vi "9_3.vi"() -> ()   [LabVIEW 2026]
panel:
  out "spreadsheet string":string
  in  "format string":string
  out "text 3":string
  in  "file path (use dialog) 4":path
  in  "file path (use dialog) 3":path
  in  "file path (use dialog) 2":path
  in  "text 2":string
  out "text":string
  in  "file path (use dialog)":path
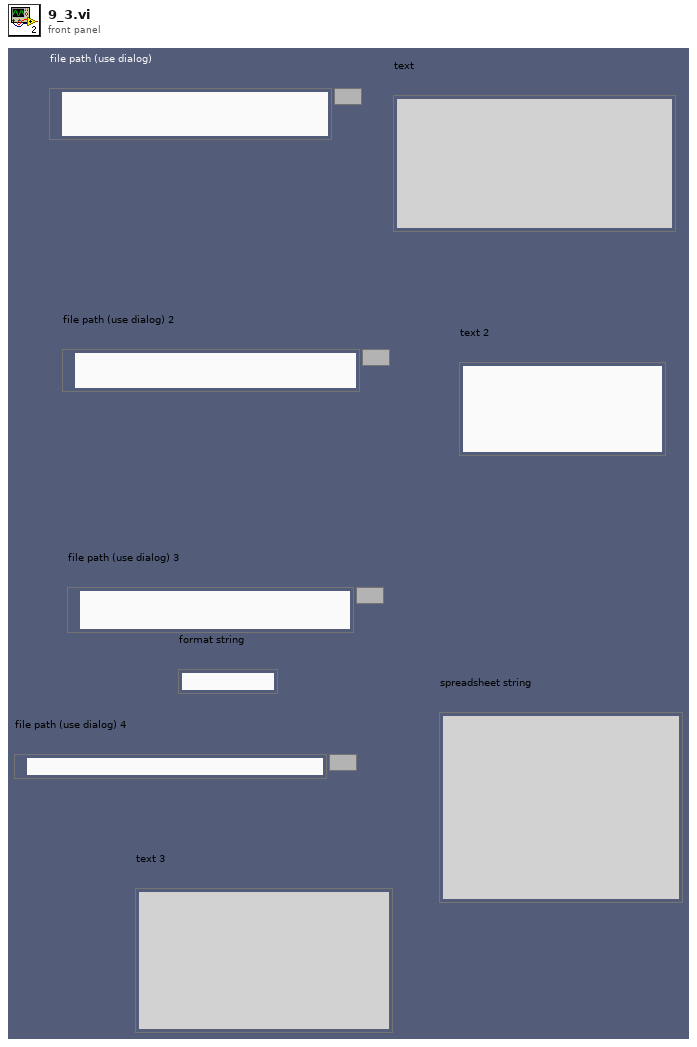
[diagram p1: front panel]
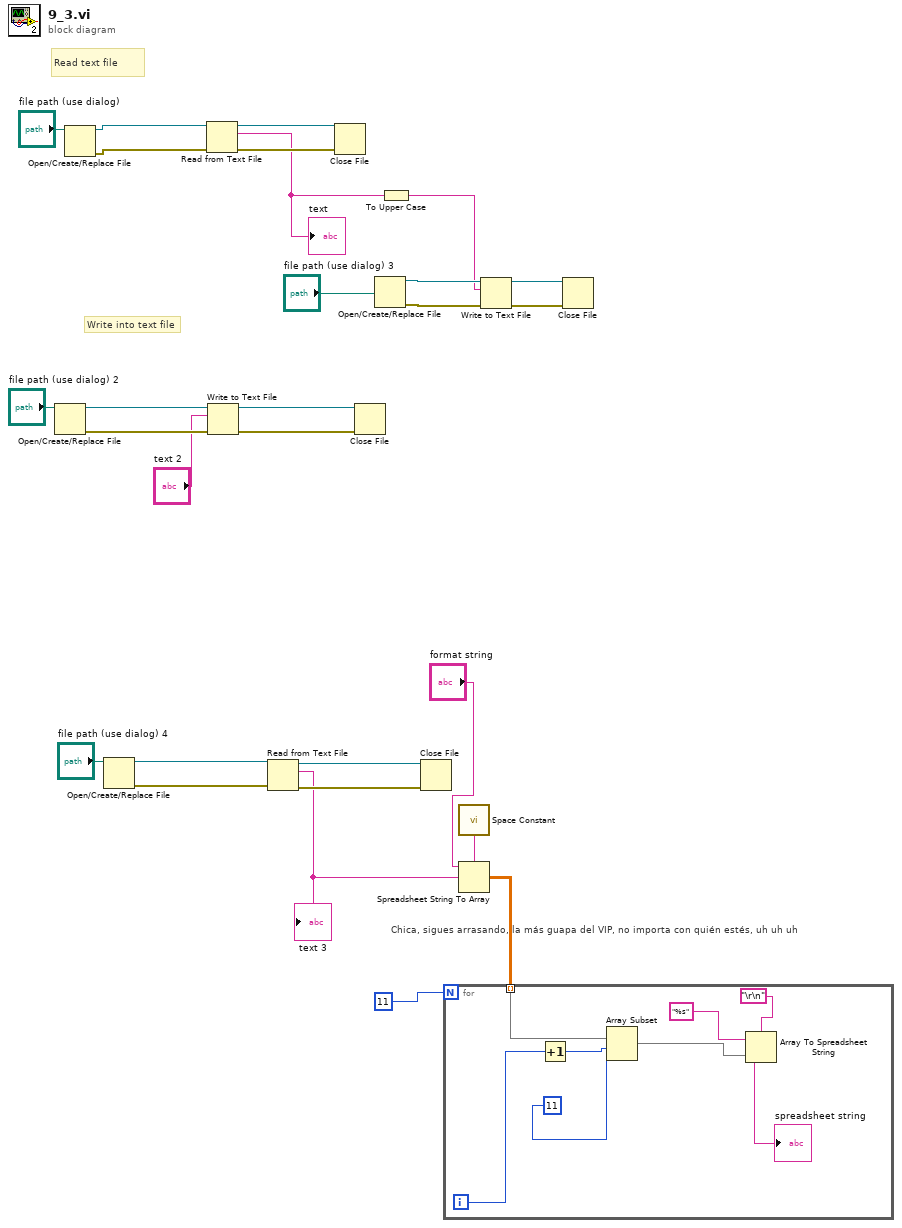
[diagram p0: block diagram]
diagram:
  # "Chica, sigues arrasando, la más guapa del VIP, no importa con quién estés, uh uh uh"
  # "Write into text file"
  # "Read text file"
  n1 = Open/Create/Replace File(file path (use dialog)="file path (use dialog) 2") -> (refnum out=w23:refnum<file>, error out=w22:errorcluster)  [unwired: 5 in, 1 out]
  n2 = Open/Create/Replace File(file path (use dialog)="file path (use dialog)") -> (refnum out=w28:refnum<file>, error out=w27:errorcluster)  [unwired: 5 in, 1 out]
  n3 = Open/Create/Replace File(file path (use dialog)="file path (use dialog) 4") -> (refnum out=w10:refnum<file>, error out=w9:errorcluster)  [unwired: 5 in, 1 out]
  n4 = Read from Text File(file (use dialog)=w28, error in=w27) -> (refnum out=w26:refnum<file>, text=w17:string, error out=w25:errorcluster)  [unwired: 2 in, 1 out]
  "text" <- w17
  n5 = Write to Text File(file (use dialog)=w23, text="text 2", error in=w22) -> (refnum out=w21:refnum<file>, error out=w20:errorcluster)  [unwired: 1 in, 1 out]
  n6 = Read from Text File(file (use dialog)=w10, error in=w9) -> (refnum out=w8:refnum<file>, text=w5:string, error out=w7:errorcluster)  [unwired: 2 in, 1 out]
  "text 3" <- w5
  n7 = Close File(refnum=w26, error in=w25) -> ()  [unwired: 2 out]
  n8 = Close File(refnum=w21, error in=w20) -> ()  [unwired: 2 out]
  n9 = Open/Create/Replace File(file path (use dialog)="file path (use dialog) 3") -> (refnum out=w16:refnum<file>, error out=w15:errorcluster)  [unwired: 5 in, 1 out]
  n10 = To Upper Case(1:w17) -> (0:w12:string)
  n11 = Close File(refnum=w8, error in=w7) -> ()  [unwired: 2 out]
  n12 = call <vilib>:"Space Constant.vi"() -> ("String"=w2:string)
  n13 = Spreadsheet String To Array(delimiter (Tab)=w2, format string="format string", spreadsheet string=w5) -> (array=w1:dbl[][])  [unwired: 1 in]
  n14 = for {
    N: 11 -> [_]
    tunnel: w1 -> [w33] mode=indexing
    i -> [w35]
    n15 = Increment(x=w35) -> (x+1=w36:i32)
    n16 = Array Subset(array=w33, index=w36, length=11) -> (w32:dbl[])
    n17 = Array To Spreadsheet String(delimiter (Tab)="\r\n", array=w32, 3:"%s" ("format string")) -> (spreadsheet string=→"spreadsheet string":string)
  }
  n18 = Write to Text File(file (use dialog)=w16, text=w12, error in=w15) -> (refnum out=w14:refnum<file>, error out=w13:errorcluster)  [unwired: 1 in, 1 out]
  n19 = Close File(refnum=w14, error in=w13) -> ()  [unwired: 2 out]
